vi "UHR-Fleezers Control (host) - Avogadro v1.vi"() -> ()   [LabVIEW 2014] (continued)
            n2226 = Bundle("Left"=w3385, "Top"=w3384, "Width"=w3383, "Height"=w3382) -> (w3373:T50)  [unwired: 1 in]
            n2227 = Bundle("Left"=w3381, "Top"=w3380, "Width"=w3379, "Height"=w3378) -> (w3372:T50)  [unwired: 1 in]
            n2228 = Bundle("Left"=w3377, "Top"=w3376, "Width"=w3375, "Height"=w3374) -> (w3371:T50)  [unwired: 1 in]
            n2229 = Build Cluster Array(w3356, w3373, w3372, w3371) -> (w3370:T51)
            n2230 = for {
              tunnel: w3392 -> [w3403]
              tunnel: w3370 -> [w3404] mode=indexing
              shift-right: [w3401] -> w3368
              shift-left: TRUE -> [w3402]
              shift-right: [w3400] -> w3366
              shift-left: _ -> [w3396]
              shift-right: [w3399] -> w3365
              shift-left: _ -> [w3395]
              shift-right: [w3398] -> w3364
              shift-left: _ -> [w3394]
              shift-right: [w3397] -> w3363
              shift-left: _ -> [w3393]
              n2231 = case shown="True" w3402 {
                selector: w3402 -> [w3409 _]
                tunnel: w3404 -> [_ w3418]
                tunnel: w3403 -> [_ w3416]
                tunnel: [w3409 w3414] -> w3401
                tunnel: [w3408 w3413] -> w3400
                tunnel: [w3407 w3412] -> w3399
                tunnel: [w3406 w3411] -> w3398
                tunnel: [w3405 w3410] -> w3397
                tunnel: w3396 -> [w3408 _]
                tunnel: w3395 -> [w3407 _]
                tunnel: w3394 -> [w3406 _]
                tunnel: w3393 -> [w3405 _]
                frame False {
                }
                frame True {
                  n2232 = Unbundle(w3418) -> (w3417:T50)
                  n2233 = call "isclickinwindow.vi"("Image Param"=w3417, "Point32"=w3416) -> ("4 Y"=w3410:i32, "3 Height"=w3411:i32, "2 X"=w3412:i32, "1 Width"=w3413:i32, "In image?"=w3415:bool)  [unwired: 1 in]
                  n2234 = Not(x=w3415) -> (.not. x?=w3414:bool)
                }
              }
            }
            n2235 = Not(x=w3368) -> (.not. x?=w3367:bool)
            n2236 = case shown="True" w3367 {
              tunnel: w3365 -> [_ w3436]
              tunnel: w3363 -> [_ w3435]
              tunnel: w3366 -> [_ w3434]
              tunnel: w3364 -> [_ w3433]
              frame False {
              }
              frame True {
                w3423 = FALSE ("Get Point")
                n2237 = local read "Scan steps (MCL)"() -> (w3419:u64)
                n2238 = local read "Actual MCL Inc (V)"() -> (w3432:dbl)
                n2239 = local read "Scan lines (y)"() -> (w3437:u64)
                n2240 = Divide "Y Pix/step"(x=w3433, y=w3437) -> (x/y=w3443:dbl)
                n2241 = Divide "X pix/step"(x=w3434, y=w3419) -> (x/y=w3441:dbl)
                n2242 = Divide "Y V/pix"(x=w3432, y=w3443) -> (x/y=w3442:dbl)
                n2243 = local read "Initial Y"() -> (w3450:dbl)
                n2244 = Divide "Y half step offset"(x=w3432, y=2.0) -> (x/y=w3421:dbl)
                n2245 = Divide "X half step offset"(x=w3432, y=2.0) -> (x/y=w3439:dbl)
                n2246 = Divide "X V/pix"(x=w3432, y=w3441) -> (x/y=w3440:dbl)
                n2247 = Multiply(x=w3435, y=w3442) -> (x*y=w3451:dbl)
                n2248 = Negate(x=w3421) -> (-x=w3444:dbl)
                n2249 = Multiply(x=w3432, y=w3419) -> (x*y=w3446:dbl)
                n2250 = Multiply(x=w3440, y=w3436) -> (x*y=w3448:dbl)
                n2251 = Negate(x=w3439) -> (-x=w3438:dbl)
                n2252 = Compound Arithmetic op=ADD(w3444, w3451, w3450) -> (w3424:dbl)
                "Pointer Y (V)" <- w3424
                n2253 = local read "Initial X"() -> (w3449:dbl)
                n2254 = Negate(x=w3448) -> (-x=w3447:dbl)
                n2255 = Compound Arithmetic op=ADD(w3438, w3446, w3449, w3447) -> (w3425:dbl)
                "Pointer X (V)" <- w3425
                n2256 = case shown="True" "Set High F Confocal Spot (X-Y)" {
                  tunnel: w3425 -> [_ w3472]
                  tunnel: w3424 -> [_ w3473]
                  frame False {
                  }
                  frame True {
                    "Confocal Y 2 (V)" <- w3473
                    "Confocal X 2 (V)" <- w3472
                  }
                }
                n2257 = local read "Scan trap 3 or Fl?"() -> (w3422:bool)
                n2258 = Or(x="Set X Only", y="Set Confocal Spot (X-Y)") -> (x .or. y?=w3428:bool)
                n2259 = Or(x="Set Confocal Spot (X-Y)", y="Set Y Only") -> (x .or. y?=w3427:bool)
                n2260 = case shown="True" w3422 {
                  tunnel: w3428 -> [w3455 w3461]
                  tunnel: w3427 -> [w3454 w3460]
                  tunnel: w3425 -> [w3453 w3458]
                  tunnel: w3424 -> [w3452 w3459]
                  frame False {
                    n2261 = case shown="True" w3454 {
                      tunnel: w3452 -> [_ w3457]
                      frame False {
                      }
                      frame True {
                        n2262 = property on="AO1" class="Slide (strict)"("Val(Sgnl)"=w3457) -> ()  [unwired: 2 in, 2 out]
                        "Confocal Y 1 (V)" <- w3457
                      }
                    }
                    n2263 = case shown="True" w3455 {
                      tunnel: w3453 -> [_ w3456]
                      frame False {
                      }
                      frame True {
                        n2264 = property on="AO2" class="Slide (strict)"("Val(Sgnl)"=w3456) -> ()  [unwired: 2 in, 2 out]
                        "Confocal X 1 (V)" <- w3456
                      }
                    }
                  }
                  frame True {
                    n2265 = case shown="True" w3460 {
                      tunnel: w3459 -> [_ w3462]
                      frame False {
                      }
                      frame True {
                        n2266 = property on="Piezo trap y\noffset (V)" class="DigNum (strict)"("Val(Sgnl)"=w3462) -> ()  [unwired: 2 in, 2 out]
                      }
                    }
                    n2267 = case shown="True" w3461 {
                      tunnel: w3458 -> [_ w3467]
                      frame False {
                      }
                      frame True {
                        n2268 = local read "AOM X Cal (nm/MHz)"() -> (w3468:dbl)
                        n2269 = local read "Trap Delta (MHz)"() -> (w3470:dbl)
                        n2270 = Subtract(x=30.0, y=w3470) -> (x-y=w3469:dbl)
                        n2271 = Multiply(x=w3469, y=w3468) -> (x*y=w3465:dbl)
                        n2272 = local read "Piezo Trap X cal (nm/V)"() -> (w3464:dbl)
                        n2273 = Divide(x=w3465, y=w3464) -> (x/y=w3463:dbl)
                        n2274 = Subtract(x=w3467, y=w3463) -> (x-y=w3466:dbl)
                        n2275 = property on="Piezo trap x\noffset (V)" class="DigNum (strict)"("Val(Sgnl)"=w3466) -> ()  [unwired: 2 in, 2 out]
                      }
                    }
                  }
                }
                n2276 = local write "Set High F Confocal Spot (X-Y)"(w3423) -> ()
                n2277 = local write "Set Confocal Spot (X-Y)"(w3423) -> ()
                n2278 = local write "Set X Only"(w3423) -> ()
                n2279 = local write "Set Y Only"(w3423) -> ()
              }
            }
          }
          frame 3 {
            n2280 = local read "BD 2 Frequency 1 (MHz)"() -> (w3475:dbl)
            n2281 = local read "BD 1 Frequency 1 (MHz)"() -> (w3476:dbl)
            n2282 = local write "Manipulating Trap"(TRUE ("Manipulating Trap")) -> ()
            n2283 = local write "Coords"(T12 {"Horizontal"=0, "Vertical"=0} ("Coords")) -> ()
            n2284 = while {
              tunnel: w3480 -> [w3485]
              tunnel: w3478 -> [w3484]
              tunnel: w3476 -> [w3483]
              tunnel: w3475 -> [w3482]
              tunnel: w3474 -> [w3481]
              stop <- w3486 stop-if-true
              n2285 = event shown="[0] \"Pane\": Mouse Move" {
                selector: _ -> [_ _]
                dyn-events: _ -> [_ _]
                timeout: _ -> [_ _]
                tunnel: ["Force Manip Abort" w3550] -> w3486
                tunnel: w3485 -> [w3493 _]
                tunnel: w3484 -> [w3491 _]
                tunnel: w3483 -> [w3490 _]
                tunnel: w3482 -> [w3489 _]
                tunnel: w3481 -> [w3487 _]
                event Mouse Move {
                  n2286 = event-data() -> ("Time"=w3494:u32, "Coords"=w3495:T12)  [unwired: 3 out]
                  n2287 = Less?(x=w3494, y=w3493) -> (x < y?=w3492:bool)
                  n2288 = case "Makes sure old motion events prior to mouse click aren't used" shown="False" w3492 {
                    tunnel: w3495 -> [w3537 _]
                    tunnel: w3491 -> [w3538 _]
                    tunnel: w3490 -> [w3512 _]
                    tunnel: w3489 -> [w3511 _]
                    tunnel: w3487 -> [w3496 _]
                    frame False {
                      n2289 = Subtract(x=w3537, y=w3538) -> (x-y=w3536:T12)
                      "Coords" <- w3536
                      n2290 = local read "Y RF Frequency Limits (MHz)"() -> (w3497:T23)
                      n2291 = To Double Precision Float(number=w3536) -> (double precision float=w3535:cluster{"Horizontal":dbl, "Vertical":dbl})
                      n2292 = Multiply(x=cluster{"Horizontal":dbl, "Vertical":dbl} {"Horizontal"=-1.0, "Vertical"=1.0}, y="Manipulation Scaling") -> (x*y=w3531:cluster{"Horizontal":dbl, "Vertical":dbl})
                      n2293 = local read "X RF Frequency Limits (MHz)"() -> (w3498:T23)
                      n2294 = Multiply(x=w3535, y=w3531) -> (x*y=w3533:cluster{"Horizontal":dbl, "Vertical":dbl})
                      n2295 = Unbundle By Name(w3533) -> ("Horizontal"=w3528:dbl, "Vertical"=w3532:dbl)
                      n2296 = Unbundle By Name(w3497) -> ("Maximum"=w3500:dbl, "Minimum"=w3499:dbl)
                      n2297 = Boolean To (0,1)(Boolean="Manip. X?") -> (0, 1=w3526:i16)
                      n2298 = Boolean To (0,1)(Boolean="Manip. Y?") -> (0, 1=w3523:i16)
                      n2299 = local read "BD 1 Frequency 2 (MHz)"() -> (w3514:dbl)
                      n2300 = Multiply(x=w3532, y=w3523) -> (x*y=w3525:dbl)
                      n2301 = Multiply(x=w3526, y=w3528) -> (x*y=w3529:dbl)
                      n2302 = local read "BD 2 Frequency 2 (MHz)"() -> (w3513:dbl)
                      n2303 = Unbundle By Name(w3498) -> ("Maximum"=w3502:dbl, "Minimum"=w3501:dbl)
                      n2304 = Add(x=w3511, y=w3525) -> (x+y=w3504:dbl)
                      n2305 = Add(x=w3512, y=w3529) -> (x+y=w3506:dbl)
                      n2306 = In Range and Coerce(upper limit=w3502, x=w3506, lower limit=w3501) -> (coerced(x)=w3505:dbl)  [unwired: 1 out]
                      n2307 = In Range and Coerce(upper limit=w3500, x=w3504, lower limit=w3499) -> (coerced(x)=w3503:dbl)  [unwired: 1 out]
                      n2308 = Subtract(x=w3505, y=w3514) -> (x-y=w3522:dbl)
                      n2309 = Subtract(x=w3503, y=w3513) -> (x-y=w3521:dbl)
                      n2310 = Square(x=w3522) -> (x^2=w3520:dbl)
                      n2311 = Square(x=w3521) -> (x^2=w3519:dbl)
                      n2312 = Add(x=w3520, y=w3519) -> (x+y=w3518:dbl)
                      n2313 = Square Root(x=w3518) -> (sqrt(x)=w3515:dbl)
                      n2314 = In Range and Coerce(upper limit="Limit Max (MHz)", x=w3515, lower limit="Limit Min (MHz)") -> (In Range?=w3508:bool)  [unwired: 1 out]
                      n2315 = Not(x="Limits Enable") -> (.not. x?=w3507:bool)
                      n2316 = Or(x=w3508, y=w3507) -> (x .or. y?=w3509:bool)
                      n2317 = case shown="True" w3509 {
                        tunnel: w3515 -> [_ w3540]
                        tunnel: w3505 -> [_ w3547]
                        tunnel: w3514 -> [_ w3546]
                        tunnel: w3503 -> [_ w3545]
                        tunnel: w3513 -> [_ w3544]
                        tunnel: w3498 -> [_ w3542]
                        tunnel: w3497 -> [_ w3541]
                        tunnel: w3496 -> [_ w3539]
                        frame False {
                        }
                        frame True {
                          n2318 = local read "BD 1 Frequency 3 (MHz)"() -> (w3548:dbl)
                          n2319 = local read "BD 2 Frequency 3 (MHz)"() -> (w3543:dbl)
                          n2320 = local write "Trap Delta (MHz)"(w3540) -> ()
                          n2321 = call "set RF board frequency - interlace.vi"("Board 2 Frequency Limits"=w3541, "Board 1 Frequency Limits"=w3542, "FPGA VI Reference In"=w3539, "Board 2 Frequency 3 (MHz)"=w3543, "Board 1 Frequency 3 (MHz)"=w3548, "Board 2 Frequency 2 (MHz)"=w3544, "Board 2 Frequency 1 (MHz)"=w3545, "Board 1 Frequency 2 (MHz)"=w3546, "Board 1 Frequency 1  (MHz)"=w3547) -> ()  [unwired: 1 in, 2 out]
                          n2322 = local write "BD 2 Frequency 1 (MHz)"(w3545) -> ()
                          n2323 = local write "BD 1 Frequency 1 (MHz)"(w3547) -> ()
                        }
                      }
                    }
                    frame True {
                    }
                  }
                }
                event Mouse Up {
                  n2324 = event-data() -> ("Button"=w3549:u16)  [unwired: 8 out]
                  n2325 = case shown="3" w3549 {
                    tunnel: [FALSE TRUE] -> w3550
                    frame 0, Default {
                    }
                    frame 3 {
                      n2326 = local read "Trap Delta (MHz)"() -> (w3552:dbl)
                      n2327 = property on="Initial delta (MHz)" class="DigNum (strict)"("Val(Sgnl)"=w3552) -> ()  [unwired: 2 in, 2 out]
                      n2328 = local write "Manipulating Trap"(FALSE ("Manipulating Trap")) -> ()
                    }
                  }
                }
              }
            }
          }
        }
      }
      event Timeout {
        n2329 = event-data() -> ()  [unwired: 4 out]
      }
      event "Stop All": Mouse Down {
        n2330 = event-data() -> ()  [unwired: 9 out]
      }
      event Mouse Move {
        n2331 = event-data() -> ()  [unwired: 6 out]
      }
    }
    n2332 = node-c288() -> ()  [unwired: 2 out]
  }
  n2333 = node-c288(w33) -> ()  [unwired: 1 out]
  n2334 = node-c288(i64 1 ("Period"), 1 ("Processor")) -> (w71:T35)  [unwired: 2 in, 2 out]
  n2335 = node-c288(3 ("Processor")) -> (w63:T35)  [unwired: 3 out]
  n2336 = timed-loop "Oscillate Trap/AOM (fishing, conjugate plane alignment)" {
    tunnel: [w3558] -> w68
    timing: w63 -> [_]
    timing-out: [_] -> w62
    tunnel: w25 -> [w3557]
    tunnel: w1 -> [w3556]
    stop <- w3558 stop-if-true
    n2337 = node-c288() -> ()  [unwired: 2 out]
    n2338 = event shown="[1] \"Fl. Triggered...\": Value Change" {
      selector: _ -> [_ _ _ _]
      dyn-events: _ -> [_ _ _ _]
      timeout: _ -> [_ _ _ _]
      tunnel: [FALSE ("Stop All") _ _ w4231] -> w3558
      tunnel: w3557 -> [w3561 _ _ _]
      tunnel: w3556 -> [_ _ w4166 _]
      event "Oscillate Set 1", "Fish for Tether": Value Change {
        n2339 = event-data() -> ()  [unwired: 6 out]
        n2340 = local read "Oscillate Set 1"() -> (w3565:bool)
        n2341 = Or(x=w3565, y="Fish for Tether") -> (x .or. y?=w3563:bool)
        n2342 = case shown="True" w3563 {
          tunnel: "Fish for Tether" -> [_ w3568]
          tunnel: w3561 -> [_ w3566]
          frame False {
          }
          frame True {
            n2343 = case shown="True" w3568 {
              selector: w3568 -> [w3571 w3577]
              tunnel: [w3571 w3577] -> w3567
              frame False {
              }
              frame True {
                n2344 = local write "Scan axis 2"(TRUE) -> ()
                n2345 = local write "Tether"(FALSE ("Tether")) -> ()
                n2346 = local read "Flow ON during cal?"() -> (w3572:bool)
                n2347 = property on="Trap Delta (MHz)" class="DigNum (strict)"("Val(Sgnl)"="Furthest Delta (MHz)") -> ()  [unwired: 2 in, 2 out]
                n2348 = Or(x="Flow ON during \nfishing?", y=w3572) -> (x .or. y?=w3573:bool)
                n2349 = Wait (ms)(milliseconds to wait=u32 500) -> ()  [unwired: 1 out]
                n2350 = property on="Sample Channel\nFlow" class="Bool (strict)"("Val(Sgnl)"=w3573) -> ()  [unwired: 2 in, 2 out]
              }
            }
            n2351 = node-c288() -> (w3570:T35)  [unwired: 1 in, 3 out]
            n2352 = timed-loop "Oscillate AOD" {
              timing: w3570 -> [_]
              timing-out: [_] -> w3569
              tunnel: w3567 -> [w3581]
              tunnel: w3566 -> [w3580]
              i -> [w3589]
              stop <- w3587 stop-if-true
              n2353 = node-c288() -> (w3588:i64)  [unwired: 1 out]
              n2354 = flat-sequence {
                tunnel: w3589 -> [w3616]
                tunnel: w3588 -> [w3615]
                tunnel: w3581 -> [w3599]
                tunnel: [w3599] -> w3586
                tunnel: [w3598] -> w3585
                tunnel: [w3597] -> w3584
                tunnel: [w3594] -> w3582
                tunnel: w3580 -> [w3590]
                tunnel: w3586 -> [w3663]
                tunnel: w3585 -> [w3661]
                tunnel: w3584 -> [w3660]
                tunnel: [w3659] -> w3583
                tunnel: w3582 -> [w3658]
                tunnel: [w3735] -> w3587
                tunnel: w3583 -> [w3734]
                frame #0 {
                  # "w (rad/s)"
                  # "t (s)"
                  n2355 = Divide(x=w3615, y=i64 1000) -> (x/y=w3591:dbl)
                  n2356 = local read "BD 1 Frequency 2 (MHz)"() -> (w3593:dbl)
                  n2357 = Multiply(x="Osc. freq. (Hz)", y=6.283185307179586) -> (x*y=w3613:dbl)
                  n2358 = Multiply(x=w3591, y=w3616) -> (x*y=w3612:dbl)
                  n2359 = Multiply(x=w3613, y=w3612) -> (x*y=w3596:dbl)
                  n2360 = local read "BD 1 Frequency 1 (MHz)"() -> (w3601:dbl)
                  n2361 = case shown="True" w3599 {
                    tunnel: w3596 -> [w3622 w3641]
                    tunnel: w3601 -> [_ w3649]
                    tunnel: w3593 -> [_ w3650]
                    tunnel: [w3619 w3645] -> w3592
                    tunnel: [FALSE w3623] -> w3597
                    tunnel: [0.0 w3637] -> w3594
                    frame False {
                      n2362 = Sine(x=w3622) -> (sin(x)=w3620:dbl)
                      n2363 = Multiply(x=w3620, y="Osc. amp. (MHz)") -> (x*y=w3619:dbl)
                    }
                    frame True {
                      # "trap position goes from 0 to 1 (0 is when it is furthest away, 1 is when closest)\nso we want to test for tether only when farther away, or x < 1"
                      # "quit if taking too long"
                      # "oscillate the trap"
                      # "Test for tether"
                      n2364 = local read "Vec Mean of T1 T2"() -> (w3626:dbl[])
                      "Trigger Signal" <- w3626
                      n2365 = Cosine(x=w3641) -> (cos(x)=w3653:dbl)
                      n2366 = Subtract(x=w3650, y=w3649) -> (x-y=w3648:dbl)
                      n2367 = Decrement(x=w3653) -> (x-1=w3652:dbl)
                      n2368 = Subtract(x=w3648, y="Closest Delta (MHz)") -> (x-y=w3646:dbl)
                      n2369 = Divide(x=w3652, y=-2.0) -> (x/y=w3636:dbl)
                      n2370 = Greater?(x=w3626, y="Stop F (pN)") -> (0:w3643:bool[])
                      n2371 = Multiply(x=w3636, y=w3646) -> (x*y=w3645:dbl)
                      n2372 = Less?(x=w3636, y="Fish mask thresh") -> (x < y?=w3635:bool)
                      n2373 = Boolean To (0,1)(Boolean=w3635) -> (0, 1=w3633:i16)
                      n2374 = Multiply(x=w3633, y=w3626) -> (x*y=w3632:dbl[])
                      n2375 = Divide(x=w3641, y=6.283185307179586) -> (x/y=w3640:dbl)
                      n2376 = Round Toward +Infinity(x=w3640) -> (ceil(x): smallest int >= x=w3637:dbl)
                      "Attempts" <- w3637
                      n2377 = Greater?(x=w3632, y="Stop F (pN) (mask)") -> (0:w3630:bool[])
                      n2378 = Or Array Elements(Boolean array=w3643) -> (logical OR=w3628:bool)
                      n2379 = Or Array Elements(Boolean array=w3630) -> (logical OR=w3627:bool)
                      n2380 = Greater?(x=w3637, y="Attempt Limit") -> (0:w3639:bool)
                      n2381 = case shown="True" w3639 {
                        frame False {
                        }
                        frame True {
                          n2382 = local write "Fish for Tether"(FALSE ("Fish for Tether")) -> ()
                          n2383 = call <vilib>:"Beep.vi"() -> ()  [unwired: 3 in, 9 out]
                          n2384 = local read "Messages"() -> (w3655:string)
                          n2385 = call "Update messages.vi"("Message to add"="Tether fishing timeout." ("Messages"), "Old message string"=w3655) -> ("New message string"=→"Messages":string)
                        }
                      }
                      n2386 = Select(t=w3628, s="Normal (on) or masked test (off)", f=w3627) -> (s? t:f=w3625:bool)
                      n2387 = And(x="Stop Fishing When Tether", y=w3625) -> (x .and. y?=w3623:bool)
                    }
                  }
                  n2388 = local read "BD 2 Frequency 1 (MHz)"() -> (w3600:dbl)
                  n2389 = Select(t=w3601, s="Scan axis 2", f=w3600) -> (s? t:f=w3604:dbl)
                  n2390 = Add(x=w3592, y=w3604) -> (x+y=w3598:dbl)
                  n2391 = Select(t=w3598, s="Scan axis 2", f=w3601) -> (s? t:f=w3607:dbl)
                  n2392 = Select(t=w3600, s="Scan axis 2", f=w3598) -> (s? t:f=w3606:dbl)
                  n2393 = local read "BD 2 Frequency 2 (MHz)"() -> (w3609:dbl)
                  n2394 = local read "BD 2 Frequency 3 (MHz)"() -> (w3608:dbl)
                  n2395 = local read "Y RF Frequency Limits (MHz)"() -> (w3602:T23)
                  n2396 = local read "X RF Frequency Limits (MHz)"() -> (w3603:T23)
                  n2397 = local read "BD 1 Frequency 3 (MHz)"() -> (w3610:dbl)
                  n2398 = call "set RF board frequency - interlace.vi"("Board 2 Frequency Limits"=w3602, "Board 1 Frequency Limits"=w3603, "FPGA VI Reference In"=w3590, "Board 2 Frequency 3 (MHz)"=w3608, "Board 1 Frequency 3 (MHz)"=w3610, "Board 2 Frequency 2 (MHz)"=w3609, "Board 2 Frequency 1 (MHz)"=w3606, "Board 1 Frequency 2 (MHz)"=w3593, "Board 1 Frequency 1  (MHz)"=w3607) -> ()  [unwired: 1 in, 2 out]
                }
                frame #1 {
                  n2399 = And(x=w3663, y=w3660) -> (x .and. y?=w3662:bool)
                  n2400 = case "Only if were fishing and now formed tether" shown="True" w3662 {
                    tunnel: w3661 -> [w3665 w3680]
                    tunnel: [w3664 w3679] -> w3659
                    tunnel: w3658 -> [_ w3675]
                    frame False {
                      n2401 = local read "Fish for Tether"() -> (w3664:bool)
                      n2402 = case shown="False" w3664 {
                        tunnel: w3665 -> [w3666 _]
                        frame False {
                          n2403 = property on="BD 1 Frequency 1 (MHz)" class="DigNum (strict)"("Val(Sgnl)"=w3666) -> ()  [unwired: 2 in, 2 out]
                        }
                        frame True {
                        }
                      }
                    }
                    frame True {
                      w3679 = FALSE ("Fish for Tether")
                      n2404 = call <vilib>:"Beep.vi"() -> ()  [unwired: 3 in, 9 out]
                      n2405 = Number To Decimal String(number=w3675, width (-)=i16 1) -> (decimal integer string=w3673:string)
                      n2406 = Concatenate Strings("Formed tether in ", w3673, " attempt(s)." ("string")) -> (w3670:string)
                      n2407 = local read "Messages"() -> (w3677:string)
                      n2408 = local write "Fish for Tether"(w3679) -> ()
                      n2409 = call "Update messages.vi"("Message to add"=w3670, "Old message string"=w3677) -> ("New message string"=w3676:string)
                      n2410 = local write "Messages"(w3676) -> ()
                      n2411 = Get Date/Time In Seconds() -> (seconds since 1Jan1904=→"Time tether formed":timestamp)
                      n2412 = local read "Flow ON during cal?"() -> (w3667:bool)
                      n2413 = property on="Sample Channel\nFlow" class="Bool (strict)"("Val(Sgnl)"=w3667) -> (error out=w3668:errorcluster)  [unwired: 2 in, 1 out]
                      n2414 = case shown="\"2\", \"3\", \"4\", \"5\", \"6\"" "Then..." {
                        selector: "Then..." -> [_ w3683]
                        tunnel: w3680 -> [w3682 _]
                        tunnel: w3668 -> [_ _]
                        frame "1", Default {
                          n2415 = property on="BD 1 Frequency 1 (MHz)" class="DigNum (strict)"("Val(Sgnl)"=w3682) -> ()  [unwired: 2 in, 2 out]
                        }
                        frame "2", "3", "4", "5", "6" {
                          n2416 = flat-sequence {
                            tunnel: w3683 -> [w3685]
                            frame #0 {
                              n2417 = property on="Trap Delta (MHz)" class="DigNum (strict)"("Val(Sgnl)"="Move to Delta 1 (MHz)") -> ()  [unwired: 2 in, 2 out]
                            }
                            frame #1 {
                              n2418 = case shown="\"5\", \"6\"" w3685 {
                                selector: w3685 -> [w3688 w3698 _]
                                frame "3", "4" {
                                n2419 = flat-sequence {
                                tunnel: w3688 -> [w3689]
                                tunnel: [w3689] -> w3686
                                tunnel: [w3691] -> w3687
                                tunnel: w3686 -> [w3691]
                                tunnel: w3687 -> [w3695]
                                frame #0 {
                                n2420 = property on="Green Laser ON" class="Bool (strict)"("Val(Sgnl)"=TRUE ("Value (Signaling)")) -> ()  [unwired: 2 in, 2 out]
                                }
                                frame #1 {
                                n2421 = Multiply(x="Wait Before Save (s)", y=u32 1000 ("x")) -> (x*y=w3693:u32)
                                n2422 = Wait (ms)(milliseconds to wait=w3693) -> ()  [unwired: 1 out]
                                }
                                frame #2 {
                                n2423 = property on="Start Saving" class="Bool (strict)"("Value"=TRUE ("Start Saving")) -> ()  [unwired: 2 in, 2 out]
                                n2424 = case shown="\"4\"" w3695 {
                                frame Default {
                                }
                                frame "4" {
                                n2425 = property on="Fl. Triggered..." class="Bool (strict)"("Val(Sgnl)"=TRUE ("Value (Signaling)")) -> ()  [unwired: 2 in, 2 out]
                                }
                                }
                                }
                                }
                                }
                                frame "5", "6" {
                                n2426 = stacked-sequence {
                                tunnel: w3698 -> [_ _ _ _ _ _ w3710]
                                frame #0 {
                                n2427 = Replace Array Subset(array=u32[] [0] ("Index Values"), new element="Raster Set Upon Tether", index=0) -> (w3699:u32[])
                                n2428 = property on="Saved AOD Raster Scan Parameter Sets" class="Arr (strict)"("Index Values"=w3699) -> ()  [unwired: 2 in, 2 out]
                                }
                                frame #1 {
                                n2429 = Wait (ms)(milliseconds to wait=u32 500) -> ()  [unwired: 1 out]
                                }
                                frame #2 {
                                n2430 = property on="Load parameters" class="Bool (strict)"("Val(Sgnl)"=TRUE ("Value (Signaling)")) -> ()  [unwired: 2 in, 2 out]
                                n2431 = case shown="True" "Green ON During Raster" {
                                frame False {
                                }
                                frame True {
                                n2432 = property on="Green Laser ON" class="Bool (strict)"("Val(Sgnl)"=TRUE ("Value (Signaling)")) -> ()  [unwired: 2 in, 2 out]
                                }
                                }
                                }
                                frame #3 {
                                n2433 = Wait (ms)(milliseconds to wait=u32 500) -> ()  [unwired: 1 out]
                                }
                                frame #4 {
                                n2434 = property on="Trap Raster Scan" class="Bool (strict)"("Val(Sgnl)"=TRUE ("Value (Signaling)")) -> ()  [unwired: 2 in, 2 out]
                                }
                                frame #5 {
                                n2435 = Wait (ms)(milliseconds to wait=u32 2000) -> ()  [unwired: 1 out]
                                }
                                frame #6 {
                                n2436 = flat-sequence {
                                tunnel: w3710 -> [w3717]
                                frame #0 {
                                n2437 = while {
                                stop <- w3713 stop-if-true
                                n2438 = local read "Raster Scanning..."() -> (w3712:bool)
                                n2439 = local read "Saving..."() -> (w3715:bool)
                                n2440 = Wait (ms)(milliseconds to wait=u32 100) -> ()  [unwired: 1 out]
                                n2441 = Not(x=w3715) -> (.not. x?=w3714:bool)
                                n2442 = Not(x=w3712) -> (.not. x?=w3711:bool)
                                n2443 = And(x=w3714, y=w3711) -> (x .and. y?=w3713:bool)
                                }
                                }
                                frame #1 {
                                n2444 = local read "Tether"() -> (w3718:bool)
                                n2445 = case shown="True" w3718 {
                                tunnel: w3717 -> [_ w3720]
                                frame False {
                                n2446 = property on="Fish for Tether" class="Bool (strict)"("Val(Sgnl)"="Fish again after \nraster break?") -> ()  [unwired: 2 in, 2 out]
                                }
                                frame True {
                                n2447 = stacked-sequence {
                                tunnel: w3720 -> [_ w3724 _ _]
                                frame #0 {
                                n2448 = property on="Trap Delta (MHz)" class="DigNum (strict)"("Val(Sgnl)"="Move to Delta 2 (MHz)") -> ()  [unwired: 2 in, 2 out]
                                n2449 = case shown="True" "Flow ON after\ntether testing?" {
                                frame False {
                                }
                                frame True {
                                n2450 = property on="Sample Channel\nFlow" class="Bool (strict)"("Val(Sgnl)"=TRUE ("Value (Signaling)")) -> ()  [unwired: 2 in, 2 out]
                                }
                                }
                                }
                                frame #1 {
                                n2451 = flat-sequence {
                                tunnel: w3724 -> [w3726]
                                frame #0 {
                                n2452 = Wait (ms)(milliseconds to wait=u32 500) -> ()  [unwired: 1 out]
                                }
                                frame #1 {
                                n2453 = case shown="\"6\"" w3726 {
                                frame Default {
                                }
                                frame "6" {
                                n2454 = property on="Green Laser ON" class="Bool (strict)"("Val(Sgnl)"=TRUE ("Green Laser ON/Interlacing")) -> ()  [unwired: 2 in, 2 out]
                                }
                                }
                                }
                                frame #2 {
                                n2455 = Wait (ms)(milliseconds to wait=u32 500) -> ()  [unwired: 1 out]
                                }
                                frame #3 {
                                n2456 = local write "Start Saving"("Save at end (5, 6)") -> ()
                                }
                                }
                                }
                                frame #2 {
                                n2457 = local read "Bead Sep. Int. Time (s)"() -> (w3732:dbl)
                                n2458 = Multiply(x=w3732, y=1000.0) -> (x*y=w3731:dbl)
                                n2459 = Wait (ms)(milliseconds to wait=w3731) -> ()  [unwired: 1 out]
                                }
                                frame #3 {
                                n2460 = property on="Remove Offset" class="Bool (strict)"("Val(Sgnl)"=TRUE ("Value (Signaling)")) -> ()  [unwired: 2 in, 2 out]
                                }
                                }
                                }
                                }
                                }
                                }
                                }
                                }
                                }
                                frame "2", Default {
                                }
                              }
                            }
                          }
                        }
                      }
                      "Tether" <- "Tether Alarm?"
                    }
                  }
                }
                frame #2 {
                  n2461 = local read "Oscillate Set 1"() -> (w3739:bool)
                  n2462 = local read "Stop All"() -> (w3737:bool)
                  n2463 = Or(x=w3739, y=w3734) -> (x .or. y?=w3736:bool)
                  n2464 = Not(x=w3736) -> (.not. x?=w3738:bool)
                  n2465 = Compound Arithmetic op=OR(w3737, w3738) -> (w3735:bool)
                }
              }
              n2466 = node-c288() -> ()  [unwired: 2 out]
            }
            n2467 = node-c288(w3569) -> ()  [unwired: 1 out]
          }
        }
      }
      event "Fl. Triggered...": Value Change {
        n2468 = event-data() -> ()  [unwired: 7 out]
        n2469 = case shown="True" "Fl. Triggered..." {
          frame False {
          }
          frame True {
            n2470 = node-c288() -> (w3750:T35)  [unwired: 4 out]
            n2471 = timed-loop {
              timing: w3750 -> [_]
              timing-out: [_] -> w3749
              tunnel: "Action" -> [w3758]
              shift-right: [w3755] -> _
              shift-left: u8 255 -> [w3757]
              shift-right: [w3752] -> _
              shift-left: 255 -> [w3754]
              stop <- w3751 stop-if-true
              # "Reset confocal spot"
              n2472 = node-c288() -> ()  [unwired: 2 out]
              n2473 = flat-sequence {
                tunnel: w3758 -> [w3778]
                tunnel: w3757 -> [w3777]
                tunnel: [w3776] -> w3756
                tunnel: w3754 -> [w3763]
                tunnel: [w3762] -> w3753
                tunnel: [w4157] -> w3751
                tunnel: w3756 -> [w4156]
                tunnel: [w4156] -> w3755
                tunnel: [w4155] -> w3752
                tunnel: w3753 -> [w4155]
                frame #0 {
                  n2474 = local read "Delta Fl. 2"() -> (w3775:dbl)
                  n2475 = local read "Delta Fl. 1"() -> (w3770:dbl)
                  n2476 = Multiply(x="Fl. Delta Thresh. (kHz)", y=1000.0) -> (x*y=w3765:dbl)
                  n2477 = Select(t=w3770, s="APD to Watch", f=w3775) -> (s? t:f=w3766:dbl)
                  n2478 = Greater?(x=w3766, y=w3765) -> (0:w3771:bool)
                  n2479 = Or(x="Force Yank", y=w3771) -> (x .or. y?=w3769:bool)
                  n2480 = And(x=w3769, y="Yank when?") -> (x .and. y?=w3767:bool)
                  n2481 = case shown="True" w3767 {
                    tunnel: w3778 -> [w3781 w3982]
                    tunnel: w3777 -> [w3783 w3978]
                    tunnel: [w3783 w3976] -> w3776
                    tunnel: w3766 -> [w3789 _]
                    tunnel: w3765 -> [w3788 _]
                    tunnel: "Force Yank" -> [w3786 _]
                    tunnel: w3763 -> [w3785 w3975]
                    tunnel: [w3784 w3975] -> w3762
                    frame False {
                      n2482 = Negate(x=w3788) -> (-x=w3780:dbl)
                      n2483 = local write "Fl. High"(TRUE ("Fl. High")) -> ()
                      n2484 = Less?(x=w3789, y=w3780) -> (x < y?=w3787:bool)
                      n2485 = Or(x=w3786, y=w3787) -> (x .or. y?=w3782:bool)
                      n2486 = case shown="True" w3782 {
                        tunnel: w3785 -> [w3790 w3800]
                        tunnel: [w3790 w3799] -> w3784
                        tunnel: w3781 -> [_ w3798]
                        frame False {
                        }
                        frame True {
                          n2487 = flat-sequence {
                            tunnel: w3800 -> [w3806]
                            tunnel: w3798 -> [w3803]
                            tunnel: [w3805] -> w3797
                            tunnel: [w3804] -> w3796
                            tunnel: [w3803] -> w3795
                            tunnel: w3794 -> [w3802]
                            tunnel: [w3802] -> w3793
                            tunnel: w3792 -> [w3801]
                            tunnel: [w3801] -> w3791
                            tunnel: [w3877] -> w3799
                            tunnel: w3797 -> [w3877]
                            tunnel: w3796 -> [w3876]
                            tunnel: w3795 -> [w3875]
                            tunnel: w3793 -> [w3874]
                            tunnel: w3791 -> [w3873]
                            frame #0 {
                              n2488 = call <vilib>:"Beep.vi"() -> ()  [unwired: 12 in]
                              n2489 = local write "Waiting"(FALSE ("Waiting")) -> ()
                              n2490 = Increment(x=w3806) -> (x+1=w3805:i32)
                              n2491 = case shown="\"Image\"" w3803 {
                                tunnel: w3805 -> [_ w3811 _]
                                frame "Alarm", Default {
                                }
                                frame "Yank" {
                                n2492 = flat-sequence {
                                tunnel: w3811 -> [w3814]
                                tunnel: [w3813] -> w3810
                                tunnel: [w3812] -> w3809
                                tunnel: w3810 -> [w3824]
                                tunnel: w3809 -> [w3825]
                                frame #0 {
                                n2493 = local read "Yank Delay (s)"() -> (w3817:dbl)
                                n2494 = local read "N Array El"() -> (w3812:u8)
                                n2495 = Quotient & Remainder(x=w3814, y=w3812) -> (x-y*floor(x/y)=w3813:i32)  [unwired: 1 out]
                                n2496 = Multiply(x=w3817, y=1000.0) -> (x*y=w3815:dbl)
                                n2497 = Wait (ms)(milliseconds to wait=w3815) -> ()  [unwired: 1 out]
                                }
                                frame #1 {
                                n2498 = local read "Yank to which?"() -> (w3819:bool)
                                n2499 = local read "Random Choice"() -> (w3829:bool)
                                n2500 = local read "Yank to Trap Delta (MHz)"() -> (w3822:dbl[])
                                n2501 = local read "Yank to SP"() -> (w3823:dbl[])
                                n2502 = Random Number (0-1)() -> (number: 0 to 1=w3828:dbl)
                                n2503 = Multiply(x=w3825, y=w3828) -> (x*y=w3827:dbl)
                                n2504 = Round Toward -Infinity(1:w3827) -> (0:w3826:dbl)
                                n2505 = Select(t=w3826, s=w3829, f=w3824) -> (s? t:f=w3820:dbl)
                                n2506 = Select(t=w3822, s=w3819, f=w3823) -> (s? t:f=w3821:dbl[])
                                n2507 = Index Array(array=w3821, index=w3820) -> (element=w3818:dbl)
                                n2508 = case shown="True" w3819 {
                                tunnel: w3818 -> [w3830 w3857]
                                frame False {
                                n2509 = flat-sequence {
                                tunnel: w3830 -> [w3831]
                                frame #0 {
                                n2510 = property on="Trap Pos FB SP" class="DigNum (strict)"("Val(Sgnl)"=w3831) -> ()  [unwired: 2 in, 2 out]
                                }
                                frame #1 {
                                n2511 = Wait (ms)(milliseconds to wait=u32 700) -> ()  [unwired: 1 out]
                                }
                                frame #2 {
                                n2512 = local read "Action (%)"() -> (w3836:dbl)
                                n2513 = Absolute Value(x=w3836) -> (abs(x)=w3835:dbl)
                                n2514 = Greater?(x=w3835, y=70.0) -> (0:w3833:bool)
                                n2515 = property on="Remove Action Offset" class="Bool (strict)"("Val(Sgnl)"=w3833) -> ()  [unwired: 2 in, 2 out]
                                }
                                frame #3 {
                                n2516 = for {
                                N: 4 -> [_]
                                n2517 = flat-sequence {
                                frame #0 {
                                n2518 = Wait (ms)(milliseconds to wait=u32 500) -> ()  [unwired: 1 out]
                                }
                                frame #1 {
                                n2519 = local read "Action (%)"() -> (w3842:dbl)
                                n2520 = Absolute Value(x=w3842) -> (abs(x)=w3841:dbl)
                                n2521 = Greater?(x=w3841, y=70.0) -> (0:w3839:bool)
                                n2522 = property on="Remove Action Offset" class="Bool (strict)"("Val(Sgnl)"=w3839) -> ()  [unwired: 2 in, 2 out]
                                }
                                }
                                }
                                }
                                frame #4 {
                                n2523 = Wait (ms)(milliseconds to wait=u32 500) -> ()  [unwired: 1 out]
                                }
                                frame #5 {
                                n2524 = local read "Mean"() -> (w3850:dbl)
                                n2525 = Greater?(x=w3850, y=11.0) -> (0:w3844:bool)
                                n2526 = Not(x=w3844) -> (.not. x?=w3845:bool)
                                n2527 = And(x=w3845, y="Shift confocal") -> (x .and. y?=w3847:bool)
                                n2528 = And(x=w3844, y="Shift confocal") -> (x .and. y?=w3848:bool)
                                n2529 = case shown="True" w3848 {
                                frame False {
                                }
                                frame True {
                                n2530 = local read "Confocal Y 2 (V)"() -> (w3854:dbl)
                                n2531 = local read "Confocal X 2 (V)"() -> (w3853:dbl)
                                n2532 = property on="AO1" class="Slide (strict)"("Val(Sgnl)"=w3854) -> ()  [unwired: 2 in, 2 out]
                                n2533 = property on="AO2" class="Slide (strict)"("Val(Sgnl)"=w3853) -> ()  [unwired: 2 in, 2 out]
                                }
                                }
                                n2534 = case shown="True" w3847 {
                                frame False {
                                }
                                frame True {
                                n2535 = local read "Confocal Y 1 (V)"() -> (w3852:dbl)
                                n2536 = local read "Confocal X 1 (V)"() -> (w3851:dbl)
                                n2537 = property on="AO1" class="Slide (strict)"("Val(Sgnl)"=w3852) -> ()  [unwired: 2 in, 2 out]
                                n2538 = property on="AO2" class="Slide (strict)"("Val(Sgnl)"=w3851) -> ()  [unwired: 2 in, 2 out]
                                }
                                }
                                }
                                frame #6 {
                                n2539 = Wait (ms)(milliseconds to wait=u32 1500) -> ()  [unwired: 1 out]
                                }
                                frame #7 {
                                n2540 = property on="Rem fb disp offset" class="Bool (strict)"("Val(Sgnl)"=TRUE ("Value (Signaling)")) -> ()  [unwired: 2 in, 2 out]
                                }
                                }
                                }
                                frame True {
                                n2541 = flat-sequence {
                                tunnel: w3857 -> [w3858]
                                frame #0 {
                                n2542 = property on="Trap Delta (MHz)" class="DigNum (strict)"("Val(Sgnl)"=w3858) -> ()  [unwired: 2 in, 2 out]
                                }
                                frame #1 {
                                n2543 = Wait (ms)(milliseconds to wait=u32 500) -> ()  [unwired: 1 out]
                                }
                                frame #2 {
                                n2544 = local read "Shift confocal"() -> (w3864:bool)
                                n2545 = local read "Mean"() -> (w3866:dbl)
                                n2546 = Greater?(x=w3866, y=11.0) -> (0:w3863:bool)
                                n2547 = Not(x=w3863) -> (.not. x?=w3862:bool)
                                n2548 = And(x=w3862, y=w3864) -> (x .and. y?=w3860:bool)
                                n2549 = And(x=w3863, y=w3864) -> (x .and. y?=w3861:bool)
                                n2550 = case shown="True" w3861 {
                                frame False {
                                }
                                frame True {
                                n2551 = local read "Confocal Y 2 (V)"() -> (w3870:dbl)
                                n2552 = local read "Confocal X 2 (V)"() -> (w3869:dbl)
                                n2553 = property on="AO2" class="Slide (strict)"("Val(Sgnl)"=w3869) -> ()  [unwired: 2 in, 2 out]
                                n2554 = property on="AO1" class="Slide (strict)"("Val(Sgnl)"=w3870) -> ()  [unwired: 2 in, 2 out]
                                }
                                }
                                n2555 = case shown="True" w3860 {
                                frame False {
                                }
                                frame True {
                                n2556 = local read "Confocal X 1 (V)"() -> (w3867:dbl)
                                n2557 = local read "Confocal Y 1 (V)"() -> (w3868:dbl)
                                n2558 = property on="AO2" class="Slide (strict)"("Val(Sgnl)"=w3867) -> ()  [unwired: 2 in, 2 out]
                                n2559 = property on="AO1" class="Slide (strict)"("Val(Sgnl)"=w3868) -> ()  [unwired: 2 in, 2 out]
                                }
                                }
                                }
                                }
                                }
                                }
                                }
                                }
                                }
                                frame "Image" {
                                n2560 = property on="Confocal Image" class="Bool (strict)"("Val(Sgnl)"=TRUE ("Value (Signaling)")) -> ()  [unwired: 2 in, 2 out]
                                }
                              }
                              n2561 = local write "Fl. High"(FALSE ("Fl. High")) -> ()
                              n2562 = local read "Time (s)"() -> (w3804:dbl)
                            }
                            frame #1 {
                              n2563 = case shown="True" "Auto F Reset" {
                                tunnel: w3876 -> [_ w3881]
                                tunnel: w3875 -> [_ w3880]
                                tunnel: w3874 -> [_ w3879]
                                tunnel: w3873 -> [_ w3878]
                                frame False {
                                }
                                frame True {
                                n2564 = node-c288() -> (w3883:T35)  [unwired: 4 in]
                                n2565 = timed-loop {
                                timing: w3883 -> [_]
                                timing-out: [_] -> w3882
                                tunnel: w3881 -> [w3888]
                                tunnel: w3880 -> [w3887]
                                tunnel: w3879 -> [w3886]
                                tunnel: w3878 -> [w3885]
                                stop <- w3884 stop-if-true
                                n2566 = node-c288() -> ()  [unwired: 1 in, 1 out]
                                n2567 = local read "Fl. Delta Thresh. (kHz)"() -> (w3897:dbl)
                                n2568 = local read "APD to Watch"() -> (w3898:bool)
                                n2569 = local read "Delta Fl. 1"() -> (w3899:dbl)
                                n2570 = local read "Delta Fl. 2"() -> (w3900:dbl)
                                n2571 = local read "Fl. Triggered..."() -> (w3891:bool)
                                n2572 = local read "Stop All"() -> (w3892:bool)
                                n2573 = local read "Reset Force"() -> (w3890:bool)
                                n2574 = Multiply(x=w3897, y=1000.0) -> (x*y=w3895:dbl)
                                n2575 = Select(t=w3899, s=w3898, f=w3900) -> (s? t:f=w3894:dbl)
                                n2576 = Not(x=w3891) -> (.not. x?=w3889:bool)
                                n2577 = Greater?(x=w3894, y=w3895) -> (0:w3893:bool)
                                n2578 = Compound Arithmetic op=OR(w3893, w3892, w3889, w3890) -> (w3884:bool)
                                n2579 = case shown="True" w3884 {
                                tunnel: w3888 -> [_ w3904]
                                tunnel: w3887 -> [_ w3908]
                                tunnel: w3886 -> [_ w3907]
                                tunnel: w3885 -> [_ w3906]
                                frame False {
                                }
                                frame True {
                                n2580 = case shown="\"Yank\"" w3908 {
                                tunnel: w3907 -> [_ w3918]
                                tunnel: w3906 -> [_ w3916]
                                frame "Image", Default {
                                }
                                frame "Yank" {
                                n2581 = flat-sequence {
                                tunnel: [w3921] -> w3919
                                tunnel: w3918 -> [w3921]
                                tunnel: [w3920] -> w3917
                                tunnel: w3916 -> [w3920]
                                tunnel: w3919 -> [w3927]
                                tunnel: w3917 -> [w3925]
                                frame #0 {
                                n2582 = local read "Yank Delay (s)"() -> (w3924:dbl)
                                n2583 = Multiply(x=w3924, y=1000.0) -> (x*y=w3922:dbl)
                                n2584 = Wait (ms)(milliseconds to wait=w3922) -> ()  [unwired: 1 out]
                                }
                                frame #1 {
                                n2585 = local read "Yank to which?"() -> (w3926:bool)